vi "UHR-Fleezers Control (host) - Avogadro v3.vi"() -> ()   [LabVIEW 2014] (continued)
          n945 = disable-structure shown="Disabled" {
            disable-tunnel: [w1522 _] -> w1520
            disable-tunnel: w1519 -> [w1521 _]
            frame Disabled {
              n946 = call-poly <vilib>:"DB Tools Open Connection.vi"("connection information"=w1521) -> ("connection reference"=w1522:T28)  [unwired: 7 in, 1 out]
            }
            frame Enabled {
            }
          }
          "connection reference" <- w1520
          n947 = local write "connection reference"(w1520) -> ()
          n948 = local write "Database link"(w1519) -> ()
        }
        frame #3 {
          # "Load active calibration to fpga"
          n949 = local read "Base N trap periods"() -> (w1524:u32)
          n950 = local read "T1 Osc Enable"() -> (w1523:bool)
          n951 = property on="T1 Osc Enable" class="Bool (strict)"("Val(Sgnl)"=w1523) -> ()  [unwired: 2 in, 2 out]
          n952 = property on="Base N trap periods" class="DigNum (strict)"("Val(Sgnl)"=w1524) -> ()  [unwired: 2 in, 2 out]
        }
      }
    }
    frame #4 {
      # "Set FIFO size and run FPGA"
      n953 = local read "FPGA error out"() -> (w1526:errorcluster)
      n954 = xnode "Invoke Method"("FPGA VI Reference In"=w1527, "error in"=w1526, "Requested Depth"="Trap AI FIFO Depth") -> ("FPGA VI Reference Out"=w1531:T41, "error out"=w1532:errorcluster)  [unwired: 1 out]
      n955 = xnode "Invoke Method"("FPGA VI Reference In"=w1531, "error in"=w1532, "Requested Depth"="Trap Position FIFO Depth") -> ("FPGA VI Reference Out"=w1529:T41, "error out"=w1528:errorcluster)  [unwired: 1 out]
      n956 = xnode "Invoke Method"("FPGA VI Reference In"=w1529, "error in"=w1528) -> ("error out"=w1525:errorcluster)  [unwired: 1 in, 1 out]
      n957 = local write "FPGA error out"(w1525) -> ()
    }
    frame #5 {
      # "Adjust FPGA timing loop phases"
      n958 = flat-sequence "Initial FPGA Loop Relative Phase Adjustment" {
        tunnel: "Initial Phase Adjustment (AI1)" -> [w1568]
        tunnel: "Initial Phase Adjustment (Vortran)" -> [w1567]
        tunnel: "Initial Phase Adj. (MCL)" -> [w1566]
        tunnel: [w1569] -> w1552
        tunnel: [w1565] -> w1551
        tunnel: "Initial Phase Adjustment (APD Acq)" -> [w1564]
        tunnel: "Initial Phase Adjustment (APD 1 Gate)" -> [w1563]
        tunnel: "Initial Phase Adjustment (Green FB)" -> [w1562]
        tunnel: "Initial Phase Adjustment (GI) 2" -> [w1561]
        tunnel: "Initial Phase Adjustment (APD 2 Gate)" -> [w1560]
        tunnel: "Initial Phase Adjustment (RI)" -> [w1559]
        tunnel: "Initial Phase Adjustment (BI DO)" -> [w1558]
        tunnel: "Initial Phase Adjustment (BI AO)" -> [w1557]
        tunnel: "Initial Phase Adjustment (APD 3 Gate)" -> [w1556]
        tunnel: w1537 -> [w1555]
        tunnel: "Initial Phase Adjustment (EMCCD Gate)" -> [w1553]
        tunnel: w1552 -> [w1571]
        tunnel: [w1572] -> w1550
        tunnel: w1551 -> [w1572]
        tunnel: [w1571] -> w1549
        tunnel: w1550 -> [w1576]
        tunnel: w1549 -> [w1575]
        tunnel: [w1574] -> w1536
        frame #0 {
          n959 = local read "FPGA error out"() -> (w1554:errorcluster)
          n960 = xnode "Read/Write Control"("FPGA VI Reference In"=w1555, "error in"=w1554, "Phase count adjustment"=w1568, "Phase count adjustment (GI)"=w1567, "Phase count adjustment (MCL)"=w1566, "Phase Count Adjustment (APD Acq)"=w1564, "Phase count adjustment (APD 1 Gate)"=w1563, "Phase count adjustment (APD 2 Gate)"=w1560, "Phase count adjustment (Green FB)"=w1562, "Phase count adjustment (GI) 2"=w1561, "Phase count adjustment (RI)"=w1559, "Phase count adjustment (BI AO)"=w1557, "Phase count adjustment (BI D)"=w1558, "Phase count adjustment (APD 3 Gate)"=w1556, "Phase Count Adjustment EMCCD Gate"=w1553) -> ("FPGA VI Reference Out"=w1565:T41, "error out"=w1569:errorcluster)
        }
        frame #1 {
          n961 = Wait (ms)(milliseconds to wait=u32 100) -> ()  [unwired: 1 out]
        }
        frame #2 {
          w1573 = TRUE
          n962 = xnode "Read/Write Control"("FPGA VI Reference In"=w1576, "error in"=w1575, "+ phase"=w1573, "+ phase (GI)"=w1573, "+ phase (MCL)"=w1573, "+ phase (APD Acq)"=w1573, "+ phase (APD 1 Gate)"=w1573, "+ phase (APD 2 Gate)"=w1573, "+ phase (Green FB)"=w1573, "+ phase (GI) 2"=w1573, "+ phase (RI)"=w1573, "+ phase (BI AO)"=w1573, "+ phase (BI D)"=w1573, "+ phase (APD 3 Gate)"=w1573, "+ phase (EMCCD Gate)"=w1573) -> ("error out"=w1574:errorcluster)  [unwired: 1 out]
        }
      }
      n963 = local write "FPGA error out"(w1536) -> ()
    }
    frame #6 {
      w1592 = 6.0  # clock mult.
      w1591 = 49152000.0  # TCXO frequ.
      w1596 = 6.0  # clock mult.
      w1597 = 49152000.0  # TCXO frequ.
      # "Added by ronen - definition of \nlimit frequencies when using dynamic feedback"
      # "Initialize trap RF synth board and set initial frequencies and amplitudes"
      n964 = local read "FPGA error out"() -> (w1577:errorcluster)
      n965 = call "set RF board frequency - interlace.vi"("Board 2 Frequency Limits"=w1603, "Board 1 Frequency Limits"=w1584, "error in"=w1577, "FPGA VI Reference In"=w1578, "Board 2 Frequency 3 (MHz)"="BD 2 Frequency 3 (MHz)", "Board 1 Frequency 3 (MHz)"="BD 1 Frequency 3 (MHz)", "Board 2 Frequency 2 (MHz)"="BD 2 Frequency 2 (MHz)", "Board 2 Frequency 1 (MHz)"="BD 2 Frequency 1 (MHz)", "Board 1 Frequency 2 (MHz)"="BD 1 Frequency 2 (MHz)", "Board 1 Frequency 1  (MHz)"="BD 1 Frequency 1 (MHz)") -> ("error out"=w1608:errorcluster, "FPGA VI Reference Out"=w1583:T41)
      n966 = Unbundle By Name(w1584) -> ("Maximum"=w1594:dbl, "Minimum"=w1585:dbl)
      n967 = call "set RF board amplitude - interlace.vi"("Board 2 Amplitude Limits"=w1605, "Board 1 Amplitude Limits"=w1604, "error in"=w1608, "FPGA VI Reference In"=w1583, "Board 2 Amplitude 3 (%)"="BD 2 Amplitude 3 (%)", "Board 1 Amplitude 3 (%)"="BD 1 Amplitude 3 (%)", "Board 2 Amplitude 2 (%)"="BD 2 Amplitude 2 (%)", "Board 2 Amplitude 1 (%)"="BD 2 Amplitude 1 (%)", "Board 1 Amplitude 2 (%)"="BD 1 Amplitude 2 (%)", "Board 1 Amplitude 1 (%)"="BD 1 Amplitude 1 (%)") -> ("error out"=w1580:errorcluster)  [unwired: 1 out]
      n968 = Multiply(x=w1585, y=1000000.0) -> (x*y=w1589:dbl)
      n969 = Multiply(x=w1594, y=1000000.0) -> (x*y=w1599:dbl)
      n970 = Scale By Power Of 2(n=48, x=w1589) -> (x*2^n=w1587:dbl)
      n971 = Subtract(x="BD 1 Frequency 1 (MHz)", y="BD 1 Frequency 2 (MHz)") -> (x-y=w1615:dbl)
      n972 = Subtract(x="BD 2 Frequency 1 (MHz)", y="BD 2 Frequency 2 (MHz)") -> (x-y=w1616:dbl)
      n973 = Scale By Power Of 2(n=48, x=w1599) -> (x*2^n=w1601:dbl)
      n974 = Multiply(x=w1591, y=w1592) -> (x*y=w1593:dbl)
      n975 = Multiply(x=w1597, y=w1596) -> (x*y=w1595:dbl)
      n976 = Square(x=w1616) -> (x^2=w1618:dbl)
      n977 = Square(x=w1615) -> (x^2=w1617:dbl)
      n978 = Divide(x=w1587, y=w1593) -> (x/y=w1588:dbl)
      n979 = Divide(x=w1601, y=w1595) -> (x/y=w1600:dbl)
      n980 = Add(x=w1617, y=w1618) -> (x+y=w1619:dbl)
      n981 = To Unsigned Quad Integer(1:w1588) -> (0:w1581:u64)
      n982 = To Unsigned Quad Integer(1:w1600) -> (0:w1582:u64)
      n983 = Square Root(x=w1619) -> (sqrt(x)=w1620:dbl)
      n984 = local write "Trap Delta (MHz)"(w1620) -> ()
      n985 = xnode "Read/Write Control"("FPGA VI Reference In"=w1583, "error in"=w1580, "FB Max Frequency"=w1582, "FB Min frequency"=w1581) -> ("error out"=w1579:errorcluster)  [unwired: 1 out]
      n986 = local write "FPGA error out"(w1579) -> ()
    }
    frame #7 {
      n987 = flat-sequence {
        frame #0 {
          n988 = local read "Trap 1 (ON/OFF)"() -> (w1625:bool)
          n989 = local write "Saving..."(FALSE ("Saving Data")) -> ()
          n990 = local write "Stop All"(FALSE ("Stop All")) -> ()
          n991 = local write "Index"(1.0 ("Index")) -> ()
          n992 = property on="Trap 1 ON" class="Bool (strict)"("Value"=w1625) -> ()  [unwired: 2 in, 2 out]
          "Manipulating Trap" <- FALSE ("Manipulating Trap")
        }
        frame #1 {
          n993 = local read "Trap 2 (ON/OFF)"() -> (w1630:bool)
          n994 = Wait (ms)(milliseconds to wait=u32 10) -> ()  [unwired: 1 out]
          n995 = property on="Trap 2 ON" class="Bool (strict)"("Val(Sgnl)"=w1630) -> ()  [unwired: 2 in, 2 out]
        }
        frame #2 {
          n996 = local read "Scan Range (nm)"() -> (w1632:dbl)
          n997 = call "Update messages.vi"("Message to add"="UHR-Fleezers ready.", "Old message string"="") -> ("New message string"=w1635:string)
          n998 = local write "Messages"(w1635) -> ()
          n999 = property on="Scan Range (nm)" class="DigNum (strict)"("Val(Sgnl)"=w1632) -> ()  [unwired: 2 in, 2 out]
        }
      }
    }
    frame #8 {
      w1666 = 0
      w1665 = 2
      w1664 = 0
      w1661 = 3
      w1660 = 2
      w1659 = 5
      w1657 = 1
      w1656 = 2
      w1698 = u32 0
      w1704 = cluster{u32, u32} {16777238, 16777238}
      w1699 = 0.0
      # "Initialize the multi-MCL offset array"
      # "Initialize valves"
      # "Cursor control of trap\n3"
      # "Graph of positions and displacements in 2D"
      n1000 = local read "MCL offset scanning range (V)"() -> (w1685:T4)
      n1001 = control-ref of="Positions \nand displacements"() -> (w1636:refnum<vi>)
      n1002 = local read "Offset file step size"() -> (w1688:dbl)
      n1003 = Divide(x=30.0, y=w1688) -> (x/y=w1679:dbl)
      n1004 = call "start_stage_trackball.vi"("Enum"=T46."Trackball XY", "Stage Controller port"=w1692) -> ("error out"=w1690:errorcluster)  [unwired: 1 in, 1 out]
      n1005 = Initialize Array(0.0, w1679) -> (w1686:dbl[])
      n1006 = call "Make Trap3 position array.vi"("MCL offset scanning range (V)"=w1685) -> ("X Data points"=w1678:u64, "Y data points"=w1681:u64)  [unwired: 3 out]
      n1007 = property on="Stage Control Serial Error" class="Clust (strict)"("Val(Sgnl)"=w1690) -> ()  [unwired: 2 in, 2 out]
      n1008 = Bundle(w1686, w1686, w1686, w1686, w1686, w1686) -> (w1683:T51)  [unwired: 1 in]
      n1009 = Multiply(x=w1681, y=w1678) -> (x*y=w1684:u64)
      n1010 = for {
        N: w1684 -> [_]
        tunnel: [w1715] -> w1682 mode=indexing
        tunnel: w1683 -> [w1715]
      }
      n1011 = Build Array("T1", "T2", "T3", "disp1", "disp2", "disp3", "junc1", "junc2", "junc3", "Mean Junc") -> (w1677:string[])
      n1012 = property class="XYGraph (strict)"(reference=w1636, "Legend:Plots Shown"=10, "XScale.Maximum"=7900.0, "XScale.Minimum"=1000.0, "YScale.Maximum"=400.0, "YScale.Minimum"=-3200.0, "Frame Color"=u32 9868950) -> (reference out=w1644:refnum<vi>)  [unwired: 1 in, 1 out]
      n1013 = Reshape Array(w1682, w1678, w1681) -> (w1680:T52)
      n1014 = local write "Multi-MCL offset array"(w1680) -> ()
      n1015 = Build Array(u32 16711680, u32 16711680, u32 16711680, u32 40779, u32 40779, u32 40779, u32 16711898, u32 16711898, u32 16711898, u32 16860) -> (w1655:u32[])
      n1016 = Build Array(w1656, w1656, w1656, w1657, w1657, w1657, w1657, w1657, w1657, w1657) -> (w1658:i32[])
      n1017 = Build Array(w1659, w1659, w1659, w1660, w1660, w1660, w1661, w1661, w1661, 5) -> (w1663:i32[])
      n1018 = Build Array(w1664, w1664, w1664, w1665, w1665, w1665, w1666, w1666, w1666, w1666) -> (w1667:i32[])
      n1019 = for {
        tunnel: w1644 -> [w1714]
        tunnel: w1655 -> [w1712] mode=indexing
        tunnel: w1658 -> [w1711] mode=indexing
        tunnel: w1663 -> [w1710] mode=indexing
        tunnel: w1667 -> [w1709] mode=indexing
        tunnel: w1677 -> [w1707] mode=indexing
        i -> [w1713]
        n1020 = property class="XYGraph (strict)"(reference=w1714, "Active Plot"=w1713) -> (reference out=w1708:refnum<vi>)  [unwired: 1 in, 1 out]
        n1021 = property class="XYGraph (strict)"(reference=w1708, "Plot.Fill/Pt. Color"=w1712, "Plot.Point Style"=w1711, "Plot.Line Width"=w1710, "Plot.Plot Interpolation"=w1709, "Plot.Plot Name"=w1707) -> ()  [unwired: 1 in, 2 out]
      }
      n1022 = control-ref of="Piezo trap cursor control"() -> (w1700:refnum<vi>)
      n1023 = property class="XYGraph (strict)"(reference=w1700, "XScale.Maximum"=10.0, "XScale.Minimum"=w1699, "YScale.Maximum"=w1699, "YScale.Minimum"=-10.0, "Plot Area Colors"=w1704, "Frame Color"=u32 9868950, "XScale.GridColors"=w1704, "YScale.GridColors"=w1704, "Cursor.Cursor Color"=u32 16711680, "Active Cursor"=w1698, "Cursor.CursorMode"=w1698) -> ()  [unwired: 1 in, 2 out]
      n1024 = call "hamilton_controller.vi"("VISA resource name in"="Visa resource for valves", "action"=T49."CONNECT") -> ("error out"=w1697:errorcluster, "VISA resource name out"=w1694:refnum<visa-resource-name>)  [unwired: 8 in]
      n1025 = call "hamilton_controller.vi"("VISA resource name in"=w1694, "error in"=w1697, "action"=T49."INITIALIZE VALVES") -> ("error out"=w1706:errorcluster)  [unwired: 7 in, 1 out]
    }
    frame #9 {
      # "Wait 5 s for all the event loops still being executed to finish."
      n1026 = Wait (ms)(milliseconds to wait=u32 5000) -> ()  [unwired: 1 out]
      n1027 = local read "FPGA error out"() -> (w1717:errorcluster)
    }
  }
  n1028 = node-c288() -> (w31:T43)  [unwired: 4 out]
  n1029 = disable-structure shown="Disabled" {
    frame Disabled {
      n1030 = while "Duncan's play event loop" {
        stop <- w1721 stop-if-true
        n1031 = Create User Event(user event datatype=TRUE ("Boolean")) -> (user event=w1722:refnum<user-event>)  [unwired: 1 in, 1 out]
        n1032 = Create User Event(user event datatype=TRUE ("Boolean")) -> (user event=w1728:refnum<user-event>)  [unwired: 1 in, 1 out]
        n1033 = global write "Global for fluorescence simulation mean (30 samples), (power series).vi" "Red Signal"(w1722) -> ()
        n1034 = global write "Global for fluorescence simulation mean (30 samples), (power series).vi" "Green Signal"(w1728) -> ()
        n1035 = register-events(w1728, w1722) -> (reference out=w1727:refnum<event-registration>)  [unwired: 2 in, 1 out]
        n1036 = event shown="[1] \"Start assembly line\": Value Change" {
          selector: w1727 -> [_ _ _ _]
          dyn-events: _ -> [_ _ _ _]
          timeout: 100 -> [_ _ _ _]
          event Timeout {
            n1037 = event-data() -> ()  [unwired: 1 in, 2 out]
          }
          event "Start assembly line": Value Change {
            n1038 = event-data() -> ("OldVal"=w1730:bool)  [unwired: 1 in, 4 out]
            n1039 = case shown="True" w1730 {
              selector: w1730 -> [_ w1731]
              frame False {
              }
              frame True {
                n1040 = property on="Move to Position 3" class="Bool (strict)"("Val(Sgnl)"=w1731) -> ()  [unwired: 2 in, 2 out]
                n1041 = case shown="1" "Numeric" {
                  frame 0, Default {
                  }
                  frame 1 {
                    n1042 = property on="Vortran Laser ON" class="Bool (strict)"("Val(Sgnl)"=TRUE ("Value (Signaling)")) -> ()  [unwired: 2 in, 2 out]
                  }
                  frame 2 {
                    n1043 = property on="Red Laser ON" class="Bool (strict)"("Val(Sgnl)"=TRUE) -> ()  [unwired: 2 in, 2 out]
                  }
                }
              }
            }
          }
          event User Event {
            n1044 = event-data() -> ("Boolean"=w1735:bool)  [unwired: 1 in, 3 out]
            "Green Fluorophore" <- w1735
            n1045 = property on="Start assembly line" class="Bool"("Val(Sgnl)"=w1735) -> ()  [unwired: 2 in, 2 out]
          }
          event User Event {
            n1046 = event-data() -> ("Boolean"=w1736:bool)  [unwired: 1 in, 3 out]
            "Red Fluorophore" <- w1736
            n1047 = property on="Start assembly line" class="Bool"("Val(Sgnl)"=w1736) -> ()  [unwired: 2 in, 2 out]
          }
        }
        n1048 = property on="Get Fluorophore" class="Bool (strict)"("Val(Sgnl)"="Get Fluorophore") -> ()  [unwired: 2 in, 2 out]
        n1049 = Wait (ms)(milliseconds to wait=u32 100) -> ()  [unwired: 1 out]
        n1050 = local read "Stop All"() -> (w1720:bool)
        n1051 = Or(x=w1720, y="stop") -> (x .or. y?=w1721:bool)
      }
    }
    frame Enabled {
    }
  }
  n1052 = timed-loop "Rough control of MCL mirror stage (debugging)" {
    tunnel: [w1739] -> w71
    timing: w31 -> [_]
    timing-out: [_] -> w30
    tunnel: w26 -> [w1737]
    stop <- w1739 stop-if-true
    n1053 = node-c288() -> ()  [unwired: 2 out]
    n1054 = case shown="1" "MCL Mode" {
      tunnel: w1737 -> [_ w1742 w1789]
      frame 0, Default {
      }
      frame 1 {
        n1055 = node-c288() -> (w1744:T43)  [unwired: 4 out]
        n1056 = timed-loop "Oscillate MCL mirror" {
          timing: w1744 -> [_]
          timing-out: [_] -> w1743
          tunnel: w1742 -> [w1745]
          i -> [w1783]
          stop <- w1746 stop-if-true
          n1057 = node-c288() -> (w1782:i64)  [unwired: 1 out]
          n1058 = Multiply(x="AO1", y=32767.0) -> (x*y=w1778:dbl)
          n1059 = Multiply(x="AO2", y=32767.0) -> (x*y=w1773:dbl)
          n1060 = Divide(x=w1778, y=10.0) -> (x/y=w1779:dbl)
          n1061 = Divide(x=w1773, y=10.0) -> (x/y=w1774:dbl)
          n1062 = To Word Integer(number=w1779) -> (16bit integer=w1771:i16)
          n1063 = To Word Integer(number=w1774) -> (16bit integer=w1770:i16)
          n1064 = Divide(x=w1782, y=i64 1000) -> (x/y=w1753:dbl)
          n1065 = Multiply(x=w1753, y=w1783) -> (x*y=w1764:dbl)
          n1066 = Multiply(x="Osc. freq. (Hz) 2", y=6.283185307179586) -> (x*y=w1765:dbl)
          n1067 = Multiply(x=w1765, y=w1764) -> (x*y=w1763:dbl)
          n1068 = Sine(x=w1763) -> (sin(x)=w1762:dbl)
          n1069 = Multiply(x=w1762, y="Osc. amp. (V)") -> (x*y=w1760:dbl)
          n1070 = Add(x=w1760, y="Osc. center (V)") -> (x+y=w1758:dbl)
          n1071 = Divide(x=w1758, y=10.0) -> (x/y=w1756:dbl)
          n1072 = Multiply(x=w1756, y=32767.0) -> (x*y=w1751:dbl)
          n1073 = Select(t=w1751, s="Scan axis", f=w1771) -> (s? t:f=w1769:dbl)
          n1074 = Select(t=w1770, s="Scan axis", f=w1751) -> (s? t:f=w1768:dbl)
          n1075 = local read "MCL Mode"() -> (w1750:u16)
          n1076 = Not Equal?(x=w1750, y=u16 1) -> (x != y?=w1747:bool)
          n1077 = local read "Stop All"() -> (w1748:bool)
          n1078 = xnode "Read/Write Control"("FPGA VI Reference In"=w1745, "AO1 (Y)"=w1769, "AO2 (X)"=w1768) -> ()  [unwired: 1 in, 2 out]
          n1079 = Compound Arithmetic op=OR(w1748, w1747) -> (w1746:bool)
          n1080 = node-c288() -> ()  [unwired: 2 out]
        }
        n1081 = node-c288(w1743) -> ()  [unwired: 1 out]
      }
      frame 2 {
        n1082 = case shown="True" "Start Scan" {
          tunnel: w1789 -> [_ w1791]
          frame False {
          }
          frame True {
            n1083 = Subtract(x="End (V)", y="Begin (V)") -> (x-y=w1798:dbl)
            n1084 = Decrement(x="N Points") -> (x-1=w1797:dbl)
            n1085 = Divide(x=w1798, y=w1797) -> (x/y=w1795:dbl)
            n1086 = for {
              N: "N Points" -> [_]
              tunnel: "Begin (V)" -> [w1814]
              tunnel: [w1806] -> w1801 mode=indexing
              tunnel: w1795 -> [w1805]
              tunnel: [w1803] -> w1794 mode=indexing
              tunnel: w1791 -> [w1802]
              i -> [w1813]
              n1087 = Multiply(x=w1805, y=w1813) -> (x*y=w1812:dbl)
              n1088 = Add(x=w1814, y=w1812) -> (x+y=w1809:dbl)
              n1089 = local read "Scan axis"() -> (w1804:bool)
              n1090 = local read "AO1"() -> (w1811:dbl)
              n1091 = local read "AO2"() -> (w1810:dbl)
              n1092 = Select(t=w1809, s=w1804, f=w1811) -> (s? t:f=w1808:dbl)
              n1093 = Select(t=w1810, s=w1804, f=w1809) -> (s? t:f=w1807:dbl)
              n1094 = flat-sequence {
                tunnel: w1808 -> [w1818]
                tunnel: w1807 -> [w1817]
                tunnel: w1802 -> [w1815]
                tunnel: [w1828] -> w1806
                tunnel: [w1827] -> w1803
                frame #0 {
                  w1821 = 10.0 ("y")
                  w1816 = 32767.0 ("y")
                  n1095 = Multiply(x=w1818, y=w1816) -> (x*y=w1824:dbl)
                  n1096 = Multiply(x=w1817, y=w1816) -> (x*y=w1822:dbl)
                  n1097 = Divide(x=w1824, y=w1821) -> (x/y=w1825:dbl)
                  n1098 = Divide(x=w1822, y=w1821) -> (x/y=w1823:dbl)
                  n1099 = To Word Integer(number=w1825) -> (16bit integer=w1819:i16)
                  n1100 = To Word Integer(number=w1823) -> (16bit integer=w1820:i16)
                  n1101 = xnode "Read/Write Control"("FPGA VI Reference In"=w1815, "AO1 (Y)"=w1819, "AO2 (X)"=w1820) -> ()  [unwired: 1 in, 2 out]
                }
                frame #1 {
                  n1102 = Wait (ms)(milliseconds to wait="DAQ Delay (ms)") -> ()  [unwired: 1 out]
                }
                frame #2 {
                  n1103 = local read "Slow mean"() -> (w1828:dbl)
                  n1104 = local read "Sigma"() -> (w1827:dbl)
                }
              }
            }
            n1105 = Bundle("Begin (V)"="Begin (V)", w1795, w1801) -> (→"MCL Scan":cluster{"Begin (V)":dbl, dbl, dbl[]})  [unwired: 1 out]
            n1106 = Bundle("Begin (V)"="Begin (V)", w1795, w1794) -> (→"MCL Scan 2":cluster{"Begin (V)":dbl, dbl, dbl[]})  [unwired: 1 out]
          }
        }
      }
    }
    n1107 = local read "Stop All"() -> (w1739:bool)
    n1108 = node-c288() -> ()  [unwired: 2 out]
  }
  n1109 = node-c288(w30) -> ()  [unwired: 1 out]
  n1110 = node-c288(2 ("Processor")) -> (w62:T43)  [unwired: 3 out]
  n1111 = timed-loop "Basic control parameters (all FPGA settings, other basic controls)" {
    shift-right: [w1836] -> _
    shift-left: errorcluster {"status"=FALSE, "code"=0, "source"=""} ("error out") -> [_]
    tunnel: [w1835] -> _
    timing: w62 -> [_]
    timing-out: [_] -> w61
    tunnel: w44 -> [w1834]
    tunnel: w40 -> [w1833]
    tunnel: w39 -> [w1832]
    tunnel: w38 -> [w1831]
    tunnel: w37 -> [w1830]
    tunnel: w26 -> [w1829]
    stop <- w1835 stop-if-true
    n1112 = node-c288() -> ()  [unwired: 2 out]
    n1113 = event shown="[22] \"Laser choice 0\", \"Laser choice 1\", \"Laser choice 2\", \"FL interlace ON count 0\", \"Fl interlace ON count 1\", \"FL interlace ON count 2\", \"FL interlace OFF count 0\", \"FL interlace OFF count 1\", \"FL interlace OFF count 2\": Value Change" {
      selector: _ -> [_ _ _ _ _ _ _ _ _ _ _ _ _ _ _ _ _ _ _ _ _ _ _ _ _ _ _ _ _ _ _ _ _ _ _ _ _ _ _ _ _ _ _ _ _ _ _ _ _ _ _ _ _ _ _ _ _ _ _ _ _ _ _ _ _ _ _ _ _ _ _ _ _ _ _ _ _ _ _ _ _ _ _ _ _ _ _ _ _ _ _ _ _ _ _ _]
      dyn-events: _ -> [_ _ _ _ _ _ _ _ _ _ _ _ _ _ _ _ _ _ _ _ _ _ _ _ _ _ _ _ _ _ _ _ _ _ _ _ _ _ _ _ _ _ _ _ _ _ _ _ _ _ _ _ _ _ _ _ _ _ _ _ _ _ _ _ _ _ _ _ _ _ _ _ _ _ _ _ _ _ _ _ _ _ _ _ _ _ _ _ _ _ _ _ _ _ _ _]
      timeout: _ -> [_ _ _ _ _ _ _ _ _ _ _ _ _ _ _ _ _ _ _ _ _ _ _ _ _ _ _ _ _ _ _ _ _ _ _ _ _ _ _ _ _ _ _ _ _ _ _ _ _ _ _ _ _ _ _ _ _ _ _ _ _ _ _ _ _ _ _ _ _ _ _ _ _ _ _ _ _ _ _ _ _ _ _ _ _ _ _ _ _ _ _ _ _ _ _ _]
      tunnel: [w1876 _ _ _ w1903 _ _ _ _ _ _ _ w2009 _ _ w2100 w2102 w2109 w2111 w2181 _ w2223 _ w2260 w2288 w2313 w2340 w2366 w2395 _ w2400 w2494 w2498 w2535 _ w2628 w2631 w2634 w2644 w2647 _ w2654 _ _ _ _ _ _ _ _ _ _ _ _ _ _ _ _ _ _ _ w3199 _ _ _ _ w3236 _ _ _ _ _ _ _ _ _ _ _ _ _ _ _ _ _ _ _ _ _ _ _ _ _ _ _ _ _] -> w1836
      tunnel: [_ _ _ _ _ _ _ _ _ _ w1988 _ _ _ _ _ _ _ _ _ _ _ _ _ _ _ _ _ _ _ _ _ _ _ _ _ _ _ _ _ _ _ _ _ _ _ _ _ _ _ _ _ _ _ _ _ _ _ _ _ _ _ _ _ _ _ _ _ _ _ _ _ _ _ _ _ _ _ _ _ _ _ _ _ _ _ _ _ _ _ _ _ _ _ _ _] -> w1835
      tunnel: [_ _ _ _ _ _ _ _ "Round T1 X" _ _ _ _ _ _ _ _ _ _ _ _ _ _ _ _ _ _ _ _ _ _ _ _ _ _ _ _ _ _ _ _ _ _ _ _ _ _ _ _ _ _ _ _ _ _ _ _ _ _ _ _ _ _ _ _ _ _ _ _ _ _ _ _ _ _ _ _ _ _ _ _ _ _ _ _ _ _ _ _ _ _ _ _ _ _ _] -> _
      tunnel: [_ _ _ "Adjust Scale\nto Mean" _ _ _ _ _ _ _ _ _ _ _ _ _ _ _ _ _ _ _ _ _ _ _ _ _ _ "Test ttrig" _ _ _ _ _ _ _ _ _ _ _ _ _ _ _ _ _ _ _ _ w2946 w3010 w3057 w3106 _ _ _ _ _ _ _ _ _ _ _ _ _ _ _ _ _ _ _ _ _ _ _ _ _ _ _ _ _ _ _ _ _ _ _ _ _ _ _ _ _] -> _
      tunnel: [_ _ _ _ _ _ _ _ _ "Round T2 X" _ "Delayed Interlace Start" _ _ _ _ _ _ _ _ _ _ _ _ _ _ _ _ _ _ _ _ _ _ _ _ _ _ _ _ _ _ _ _ _ _ _ _ _ _ _ _ _ _ _ _ _ _ _ _ _ _ _ _ _ _ _ _ _ _ _ _ _ _ _ _ _ _ _ _ _ _ _ _ _ _ _ _ _ _ _ _ _ _ _ _] -> _
      tunnel: w1834 -> [_ _ _ _ _ _ _ _ _ _ _ _ _ _ _ _ _ _ _ _ _ _ _ _ _ _ _ _ _ _ _ _ _ _ _ _ _ _ _ _ _ _ _ _ _ _ _ w2916 w2924 w2931 w2937 w2945 _ _ w3105 _ _ _ _ _ _ _ _ _ _ _ _ _ _ _ _ _ _ _ _ _ _ _ _ _ _ _ _ _ _ _ _ _ _ _ _ _ _ _ _ _]
      tunnel: w1833 -> [_ _ _ _ _ _ _ _ _ _ _ _ _ _ _ _ _ _ _ _ _ _ _ _ _ _ _ _ _ _ _ _ _ _ _ _ _ _ _ _ _ _ _ _ _ w2803 _ _ _ _ _ _ w3009 _ _ w3112 _ w3124 _ w3140 _ _ _ _ _ _ _ _ _ _ _ _ _ _ _ _ _ _ _ _ _ _ _ _ _ _ _ _ _ _ _ _ _ _ _ _]
      tunnel: w1832 -> [_ _ _ _ _ _ _ _ _ _ _ _ _ _ _ _ _ _ _ _ _ _ _ _ _ _ _ _ _ _ _ _ _ _ _ _ _ _ _ _ _ _ _ _ _ _ _ _ _ _ _ _ _ _ _ _ _ _ _ _ _ _ _ _ _ _ _ _ _ _ _ _ _ _ _ _ _ _ _ _ _ _ _ _ _ _ _ _ _ _ _ _ _ _ _ _]
      tunnel: w1831 -> [_ _ _ _ _ _ _ _ _ _ _ _ _ _ _ _ _ _ _ _ _ _ _ _ _ _ _ _ _ _ _ _ _ _ _ _ _ _ _ _ _ _ w2665 _ _ _ _ _ _ _ _ _ _ w3056 _ _ w3118 _ w3132 _ w3166 _ _ _ _ _ _ _ _ _ _ _ _ _ _ _ _ _ _ _ _ _ _ _ _ _ _ _ _ _ _ _ _ _ _ _]
      tunnel: w1830 -> [_ _ _ _ _ _ _ _ _ _ _ _ _ _ _ _ _ _ _ _ _ _ _ _ _ _ _ _ _ _ _ _ _ _ _ _ _ _ _ _ _ _ _ _ _ _ _ _ _ _ _ _ _ _ _ _ _ _ _ _ _ _ _ _ _ _ _ _ _ _ _ _ _ _ _ _ _ _ _ _ _ _ _ _ _ _ _ _ _ _ _ _ _ _ _ _]
      tunnel: w1829 -> [w1839 _ _ _ w1902 _ w1928 _ _ _ _ _ w2000 _ _ w2084 w2101 w2108 w2110 w2146 _ w2212 w2247 w2258 w2270 w2295 w2323 w2343 w2371 w2396 w2398 w2402 w2495 w2499 _ w2625 w2629 w2632 w2642 w2645 _ w2653 _ _ w2748 _ _ _ _ _ _ _ _ _ _ _ _ _ _ _ _ w3192 _ w3213 _ w3220 w3235 _ w3242 w3269 w3276 w3292 w3300 _ w3311 _ w3355 _ _ w3409 w3440 w3444 w3452 _ w3516 w3526 w3545 _ _ _ _ _ _ w3698 w3703 w3710]
      tunnel: [_ _ _ _ _ _ _ _ _ _ w1987 _ _ _ _ _ _ _ _ _ _ _ _ _ _ _ _ _ _ _ _ _ _ _ _ _ _ _ _ _ _ _ _ w2745 w2750 _ _ _ _ _ _ _ _ _ _ _ _ _ _ _ _ _ _ _ _ _ _ _ _ _ _ _ _ _ _ _ _ _ _ _ _ _ _ _ _ _ _ _ _ _ _ _ _ _ _ _] -> _
      event "AI Count (ticks)", "Sets to FIFO (Traps)", "Save ave N", "FPGA Ave.", "# Samples/channel", "N sets to save": Value Change {
        # "RG 18-01-16 Increased amount of elements to read for trap position, to add x and y for piezo trap"
        # "So that if 'Save ave N' is updated, the AOD scanning code updates too."
        n1114 = event-data() -> ()  [unwired: 6 out]
        n1115 = local read "AI Count (ticks)"() -> (w1860:u16)
        n1116 = Divide(x=40000000.0, y=w1860) -> (x/y=w1852:dbl)
        "AI rate (Hz)" <- w1852
        "Ave. Rate (Hz)" <- w1852
        n1117 = Reciprocal(x=w1852) -> (1/x=→"Ave. Period (s)":dbl)
        n1118 = Unbundle By Name("Sets to FIFO (Traps)") -> ("Set 1"=w1843:bool, "Set 2"=w1842:bool, "Set 3"=w1841:bool)
        n1119 = Divide(x=w1852, y="N Acq Sets (Traps + Fl.)") -> (x/y=w1873:dbl)
        "Data Rate (Hz)" <- w1873
        n1120 = Reciprocal(x=w1873) -> (1/x=→"Data Period (s)":dbl)
        n1121 = Boolean To (0,1)(Boolean="Sets to FIFO (Traps)") -> (0, 1=w1868:cluster{"Set 1":i16, "Set 2":i16, "Set 3":i16})
        n1122 = xnode "Read/Write Control"("FPGA VI Reference In"=w1839, "ai count"=w1860, "Set 1"=w1843, "Set 2"=w1842, "Set 3"=w1841, "N of AI1 Int Acq Sets"="N Acq Sets (Traps + Fl.)") -> ("error out"=w1876:errorcluster)  [unwired: 1 in, 1 out]
        n1123 = Cluster To Array(cluster=w1868) -> (array=w1867:i16[])
        n1124 = local read "Save ave N"() -> (w1872:dbl)
        n1125 = To Unsigned Long Integer(number=w1867) -> (unsigned 32bit integer=w1849:u32[])
        n1126 = Multiply(x=w1860, y="N Acq Sets (Traps + Fl.)") -> (x*y=w1858:u16)
        n1127 = local read "Scan steps (AOD)"() -> (w1869:u64)
        n1128 = Add Array Elements(numeric array=w1849) -> (sum=w1861:u32)
        "Trap Sets" <- w1861
        n1129 = Divide(x=w1873, y=w1872) -> (x/y=w1871:dbl)
        "Save Data Rate (Hz)" <- w1871
        n1130 = Reciprocal(x=w1871) -> (1/x=→"Save Data Period (s)":dbl)
        n1131 = property on="Scan steps (AOD)" class="DigNum (strict)"("Val(Sgnl)"=w1869) -> ()  [unwired: 2 in, 2 out]
        n1132 = Multiply(x=w1858, y="# Samples/trap") -> (x*y=w1856:u32)
        "Counts/DMA" <- w1856
        n1133 = property on="Trap Disp. Downsample" class="DigNum (strict)"("Maximum"="# Samples/trap") -> ()  [unwired: 2 in, 2 out]
        n1134 = Multiply(x=w1861, y="# Samples/trap") -> (x*y=w1850:u32)
        "# Samples/channel" <- w1850
        n1135 = Multiply(x=w1850, y=u32 8) -> (x*y=→"Trap AI Elements/DMA read":u32)
        n1136 = local read "APD Int. Count"() -> (w1857:u32)
        n1137 = Multiply(x=w1850, y=u32 5) -> (x*y=→"Trap Pos Elements/DMA read":u32)
        n1138 = Divide(x=w1856, y=w1857) -> (x/y=w1847:dbl)
        "APD Samples/FIFO Acq." <- w1847
        n1139 = Divide(x=w1856, y=40000000.0) -> (x/y=w1854:dbl)
        "DMA Update Period (s)" <- w1854
        n1140 = local read "Number of APDs"() -> (w1840:u8)
        n1141 = Multiply(x=w1840, y=w1847) -> (x*y=→"APD Elements/DMA read":dbl)
        n1142 = property on="APD Disp. Downsample" class="DigNum (strict)"("Maximum"=w1847) -> ()  [unwired: 2 in, 2 out]
        n1143 = local read "N sets to save"() -> (w1866:u32)
        n1144 = Multiply(x=w1854, y=w1866) -> (x*y=→"Total Time (s) 2":dbl)
        "FPGA Averaging" <- FALSE ("FPGA Averaging")
      }
      event "Remove Offset": Value Change {
        n1145 = event-data() -> ()  [unwired: 7 out]
        n1146 = local write "Remove Offset"(FALSE ("Remove Offset")) -> ()
        n1147 = local read "Bead Mean (nm)"() -> (w1878:dbl)
        n1148 = local read "Offset (nm)"() -> (w1879:dbl)
        n1149 = Add(x=w1878, y=w1879) -> (x+y=w1877:dbl)
        n1150 = local write "Offset (nm)"(w1877) -> ()
      }
      event "Detector Type": Value Change {
        n1151 = event-data() -> ()  [unwired: 7 out]
        n1152 = local read "AI labels"() -> (w1883:string[])
        n1153 = property on="High Res. Display" class="Ring (strict)"("Strings []"=w1883) -> ()  [unwired: 2 in, 2 out]
        n1154 = Build Array (concatenate)(w1883, "none") -> (w1884:string[])
        n1155 = property on="FFT 1 Choice 1" class="Ring (strict)"("Strings []"=w1884) -> ()  [unwired: 2 in, 2 out]
        n1156 = property on="FFT 1 Choice 2" class="Ring (strict)"("Strings []"=w1884) -> ()  [unwired: 2 in, 2 out]
        n1157 = property on="FFT 2 Choice 1" class="Ring (strict)"("Strings []"=w1884) -> ()  [unwired: 2 in, 2 out]
        n1158 = property on="FFT 2 Choice 2" class="Ring (strict)"("Strings []"=w1884) -> ()  [unwired: 2 in, 2 out]
        n1159 = Bundle("APD 1", "APD 2", "APD 3") -> (w1887:cluster{string, string, string})  [unwired: 1 out]
        n1160 = Cluster To Array(cluster=w1887) -> (array=w1885:string[])
        n1161 = Build Array (concatenate)(w1885, w1884) -> (w1889:string[])
        n1162 = Array Size(array=w1889) -> (size(s)=w1881:i32)
        n1163 = property on="Signals to Plot" class="LstBox (strict)"("Item Names"=w1889) -> ()  [unwired: 2 in, 2 out]
        n1164 = property on="Signals to Plot" class="LstBox (strict)"("Number of Rows"=w1881) -> ()  [unwired: 2 in, 2 out]
        n1165 = property on="All Signals" class="WFChart (strict)"("LegNumRows"=w1881) -> ()  [unwired: 2 in, 2 out]
      }
      event "Adjust Scale\nto Mean": Value Change {
        n1166 = event-data() -> ()  [unwired: 7 out]
        n1167 = local read "APD rates cluster"() -> (w1892:T2)
        n1168 = Unbundle By Name(w1892) -> ("APD 1 Rate (Hz)"=w1891:dbl)
        n1169 = Multiply(x=1000.0, y="Above (kHz)") -> (x*y=w1898:dbl)
        n1170 = Multiply(x=1000.0, y="Below (kHz)") -> (x*y=w1896:dbl)
        n1171 = Add(x=w1898, y=w1891) -> (x+y=w1893:dbl)
        n1172 = Subtract(x=w1891, y=w1896) -> (x-y=w1894:dbl)
        n1173 = property on="APD Chart" class="WFChart (strict)"("YScale.Minimum"=w1894) -> ()  [unwired: 2 in, 2 out]
        n1174 = property on="APD Chart" class="WFChart (strict)"("YScale.Maximum"=w1893) -> ()  [unwired: 2 in, 2 out]
      }
      event "Phase adj. (AI1)", "+ phase (AI1)", "- phase (AI1)": Value Change {
        n1175 = event-data() -> ()  [unwired: 7 out]
        n1176 = Negate(x="Phase adj. (AI1)") -> (-x=w1910:i16)
        n1177 = Select(t=w1910, s="- phase (AI1)", f="Phase adj. (AI1)") -> (s? t:f=w1909:i16)
        n1178 = xnode "Read/Write Control"("FPGA VI Reference In"=w1902, "Phase count adjustment"=w1909) -> ("FPGA VI Reference Out"=w1908:T41, "error out"=w1907:errorcluster)  [unwired: 2 in]
        n1179 = Or(x="- phase (AI1)", y="+ phase (AI1)") -> (x .or. y?=w1904:bool)
        n1180 = xnode "Read/Write Control"("FPGA VI Reference In"=w1908, "error in"=w1907, "+ phase"=w1904) -> ("error out"=w1903:errorcluster)  [unwired: 1 in, 1 out]
      }
      event "Signals to Plot": Double Click {
        w1922 = u32 9868950 ("Color Box")
        n1181 = event-data() -> ("Row"=w1913:i32)  [unwired: 9 out]
        n1182 = property on="All Signals" class="WFChart (strict)"("Active Plot"=w1913) -> (error out=w1912:errorcluster)  [unwired: 2 in, 1 out]
        n1183 = property on="All Signals" class="WFChart (strict)" props=["Plot", "Plot Color", "Plot", "Visible?"](error in=w1912) -> (error out=w1915:errorcluster, "Plot.Visible?"=w1914:bool)  [unwired: 1 in, 2 out]
        n1184 = Select(t=FALSE ("Plot.Visible"), s=w1914, f=TRUE ("Plot.Visible")) -> (s? t:f=w1917:bool)
        n1185 = property on="All Signals" class="WFChart (strict)"(error in=w1915, "Plot.Visible?"=w1917) -> (error out=w1916:errorcluster)  [unwired: 1 in, 1 out]
        n1186 = property on="All Signals" class="WFChart (strict)"(error in=w1916) -> (error out=w1918:errorcluster, "Plot.Plot Color"=w1919:u32)  [unwired: 1 in, 1 out]
        n1187 = property on="Signals to Plot" class="LstBox (strict)"(error in=w1918, "Active Row"=w1913) -> (error out=w1923:errorcluster)  [unwired: 1 in, 1 out]
        n1188 = Select(t=w1919, s=w1917, f=u32 0) -> (s? t:f=w1924:u32)
        n1189 = property on="Signals to Plot" class="LstBox (strict)"(error in=w1923, "CellFontColor"=w1924, "SelColor"=w1922, "CellBG"=w1922, "CellFontSize"=u32 20 ("Active Row:Cell Font:Size"), "CellFontBold"=TRUE ("Active Row:Cell Font:Bold")) -> ()  [unwired: 1 in, 2 out]
      }
      event "BD 1 Frequency 1 (MHz)", "BD 1 Frequency 2 (MHz)", "BD 1 Frequency 3 (MHz)", "BD 2 Frequency 1 (MHz)", "BD 2 Frequency 2 (MHz)", "BD 2 Frequency 3 (MHz)", "Trap Delta (MHz)", "Update all trap values": Value Change {
        # "This is so you can set trap frequencies\nvia local variables and then update\nall at once"
        n1190 = event-data() -> ("CtlRef"=w1932:refnum<vi>)  [unwired: 6 out]
        n1191 = control-ref of="Trap Delta (MHz)"() -> (w1931:refnum<vi>)
        n1192 = Equal?(x=w1931, y=w1932) -> (x = y?=w1930:bool)
        n1193 = local write "Update all trap values"(FALSE ("Update all trap values")) -> ()
        n1194 = case shown="False" "Oscillate Set 1" {
          tunnel: w1930 -> [w1946 _]
          tunnel: w1928 -> [w1944 _]
          frame False {
            n1195 = local read "BD 1 Frequency 2 (MHz)"() -> (w1942:dbl)
            n1196 = case shown="True" "Symmetric \nmanual\n motion" {
              tunnel: "Trap Delta (MHz)" -> [w1968 w1975]
              tunnel: [w1969 w1973] -> w1934
              tunnel: [w1967 w1971] -> w1936
              tunnel: w1942 -> [w1969 _]
              frame False {
                n1197 = Subtract(x=w1969, y=w1968) -> (x-y=w1967:dbl)
              }
              frame True {
                n1198 = Divide(x=w1975, y=2.0) -> (x/y=w1972:dbl)
                n1199 = Add(x=w1972, y="center Hz for  manual\nsymmetric motion") -> (x+y=w1973:dbl)
                n1200 = Subtract(x="center Hz for  manual\nsymmetric motion", y=w1972) -> (x-y=w1971:dbl)
              }
            }
            n1201 = local read "BD 1 Frequency 1 (MHz)"() -> (w1937:dbl)
            n1202 = Not(x="Symmetric \nmanual\n motion") -> (.not. x?=w1940:bool)
            n1203 = And(x=w1940, y="move Con X?") -> (x .and. y?=w1938:bool)
            n1204 = Subtract(x=w1937, y=w1936) -> (x-y=w1935:dbl)
            n1205 = Select(t=w1936, s=w1946, f=w1937) -> (s? t:f=w1945:dbl)
            n1206 = local read "Y RF Frequency Limits (MHz)"() -> (w1947:T27)
            n1207 = case shown="True" w1938 {
              tunnel: w1935 -> [_ w1966]
              frame False {
              }
              frame True {
                n1208 = property on="AOM X Cal (nm/MHz)" class="DigNum (strict)"() -> ("Value"=w1965:dbl)  [unwired: 2 in, 2 out]
                n1209 = property on="MCL Step Position Ratio" class="DigNum (strict)"() -> ("Value"=w1959:dbl)  [unwired: 2 in, 2 out]
                n1210 = Compound Arithmetic op=MULTIPLY(w1966, w1965, w1959) -> (w1964:dbl)
                n1211 = property on="MCL X Cal (nm/V)" class="DigNum (strict)"() -> ("Value"=w1963:dbl)  [unwired: 2 in, 2 out]
                n1212 = Divide(x=w1964, y=w1963) -> (x/y=w1962:dbl)
                n1213 = property on="AO2" class="Slide (strict)"() -> ("Value"=w1961:dbl)  [unwired: 2 in, 2 out]
                n1214 = Add(x=w1962, y=w1961) -> (x+y=w1960:dbl)
                n1215 = property on="AO2" class="Slide (strict)"("Val(Sgnl)"=w1960) -> ()  [unwired: 2 in, 2 out]
              }
            }
            n1216 = local read "X RF Frequency Limits (MHz)"() -> (w1948:T27)
            n1217 = local write "BD 1 Frequency 1 (MHz)"(w1945) -> ()
            n1218 = local read "BD 1 Frequency 3 (MHz)"() -> (w1957:dbl)
            n1219 = local read "BD 2 Frequency 1 (MHz)"() -> (w1951:dbl)
            n1220 = local read "BD 2 Frequency 2 (MHz)"() -> (w1950:dbl)
            n1221 = local read "BD 2 Frequency 3 (MHz)"() -> (w1958:dbl)
            n1222 = call "set RF board frequency - interlace.vi"("Board 2 Frequency Limits"=w1947, "Board 1 Frequency Limits"=w1948, "FPGA VI Reference In"=w1944, "Board 2 Frequency 3 (MHz)"=w1958, "Board 1 Frequency 3 (MHz)"=w1957, "Board 2 Frequency 2 (MHz)"=w1950, "Board 2 Frequency 1 (MHz)"=w1951, "Board 1 Frequency 2 (MHz)"=w1934, "Board 1 Frequency 1  (MHz)"=w1945) -> ()  [unwired: 1 in, 2 out]
            n1223 = Subtract(x=w1951, y=w1950) -> (x-y=w1955:dbl)
            n1224 = local write "BD 1 Frequency 2 (MHz)"(w1934) -> ()
            n1225 = Subtract(x=w1945, y=w1934) -> (x-y=w1956:dbl)
            n1226 = Square(x=w1955) -> (x^2=w1953:dbl)
            n1227 = Square(x=w1956) -> (x^2=w1954:dbl)
            n1228 = Add(x=w1954, y=w1953) -> (x+y=w1952:dbl)
            n1229 = Square Root(x=w1952) -> (sqrt(x)=w1949:dbl)
            n1230 = property on="Initial delta (MHz)" class="DigNum (strict)"("Val(Sgnl)"=w1949) -> ()  [unwired: 2 in, 2 out]
            n1231 = local write "Trap Delta (MHz)"(w1949) -> ()
          }
          frame True {
          }
        }
      }
      event "manual raster set": Value Change {
        n1232 = event-data() -> ()  [unwired: 7 out]
        n1233 = flat-sequence {
          frame #0 {
            n1234 = Replace Array Subset(array=u32[] [0] ("Index Values"), new element="manual raster set", index=0) -> (w1976:u32[])
            n1235 = property on="Saved AOD Raster Scan Parameter Sets" class="Arr (strict)"("Index Values"=w1976) -> ()  [unwired: 2 in, 2 out]
          }
          frame #1 {
            n1236 = property on="Load parameters" class="Bool (strict)"("Val(Sgnl)"=TRUE ("Value (Signaling)")) -> ()  [unwired: 2 in, 2 out]
          }
        }
      }
      event "Round T1 X": Value Change {
        n1237 = event-data() -> ()  [unwired: 7 out]
        n1238 = local read "BD 1 Frequency 1 (MHz)"() -> (w1983:dbl)
        n1239 = Round To Nearest(number=w1983) -> (nearest integer value=w1982:dbl)
        n1240 = property on="BD 1 Frequency 1 (MHz)" class="DigNum (strict)"("Val(Sgnl)"=w1982) -> ()  [unwired: 2 in, 2 out]
      }
      event "Round T2 X": Value Change {
        n1241 = event-data() -> ()  [unwired: 7 out]
        n1242 = local read "BD 1 Frequency 2 (MHz)"() -> (w1985:dbl)
        n1243 = Round To Nearest(number=w1985) -> (nearest integer value=w1984:dbl)
        n1244 = property on="BD 1 Frequency 2 (MHz)" class="DigNum (strict)"("Val(Sgnl)"=w1984) -> ()  [unwired: 2 in, 2 out]
      }
      event "Stop All": Value Change {
        n1245 = event-data() -> ()  [unwired: 7 out]
        n1246 = flat-sequence {
          tunnel: [w1991] -> w1989
          tunnel: [w1994] -> w1987
          tunnel: w1989 -> [w1994]
          tunnel: [TRUE] -> w1988
          frame #0 {
            n1247 = local read "Visa resource for valves"() -> (w1990:refnum<visa-resource-name>)
            n1248 = call "hamilton_controller.vi"("VISA resource name in"=w1990, "action"=T49."DISCONNECT") -> ("error out"=w1991:errorcluster)  [unwired: 8 in, 1 out]
          }
          frame #1 {
          }
        }
      }
      event "Delayed Interlace Start": Value Change {
        n1249 = event-data() -> ()  [unwired: 7 out]
        n1250 = flat-sequence {
          frame #0 {
            n1251 = Multiply(x="Delay to Interlace (s)", y=1000.0) -> (x*y=w1996:dbl)
            n1252 = Wait (ms)(milliseconds to wait=w1996) -> ()  [unwired: 1 out]
          }
          frame #1 {
            n1253 = property on="Laser interlacing mode" class="RadioBtnsControl (strict)"("Val(Sgnl)"=enum32{"Laser ON", "Laser OFF", "Interlace"}."Interlace" ("Value (Signaling)")) -> ()  [unwired: 2 in, 2 out]
          }
        }
      }
      event "BD 1 Amplitude 1 (%)", "BD 1 Amplitude 2 (%)", "BD 1 Amplitude 3 (%)", "BD 2 Amplitude 1 (%)", "BD 2 Amplitude 2 (%)", "BD 2 Amplitude 3 (%)", "Trap 1 ON", "Trap 2 ON", "Trap 3 ON", "Feedback On/Off", "All FB On/Off": Value Change {
        w2021 = i16 1 ("f")
        n1254 = event-data() -> ()  [unwired: 7 out]
        n1255 = local write "Trap 1 (ON/OFF)"("Trap 1 ON") -> ()
        n1256 = local write "Trap 2 (ON/OFF)"("Trap 2 ON") -> ()
        n1257 = Boolean To (0,1)(Boolean="Trap 3 ON") -> (0, 1=w2022:i16)
        n1258 = Boolean To (0,1)(Boolean="Trap 1 ON") -> (0, 1=w2023:i16)
        n1259 = Boolean To (0,1)(Boolean="Trap 2 ON") -> (0, 1=w2024:i16)
        n1260 = Select(t=w2024, s="Trap ON/OFF X or Y Amp?", f=w2021) -> (s? t:f=w2019:i16)
        n1261 = Select(t=w2023, s="Trap ON/OFF X or Y Amp?", f=w2021) -> (s? t:f=w2020:i16)
        n1262 = Select(t=w2022, s="Trap ON/OFF X or Y Amp?", f=w2021) -> (s? t:f=w2018:i16)
        n1263 = Select(t=w2021, s="Trap ON/OFF X or Y Amp?", f=w2024) -> (s? t:f=w2016:i16)
        n1264 = Select(t=w2021, s="Trap ON/OFF X or Y Amp?", f=w2023) -> (s? t:f=w2017:i16)
        n1265 = Select(t=w2021, s="Trap ON/OFF X or Y Amp?", f=w2022) -> (s? t:f=w2015:i16)
        n1266 = And(x="All FB On/Off", y="Feedback On/Off") -> (x .and. y?=w2013:cluster{"Set 1":bool, "Set 2":bool})
        n1267 = local read "BD 1 Amplitude 1 (%)"() -> (w2031:dbl)
        n1268 = local read "BD 1 Amplitude 2 (%)"() -> (w2030:dbl)
        n1269 = local read "BD 1 Amplitude 3 (%)"() -> (w2029:dbl)
        n1270 = Unbundle By Name(w2013) -> ("Set 1"=w2008:bool, "Set 2"=w2005:bool)
        n1271 = local read "Y RF Amplitude Limits (%)"() -> (w2001:T27)
        n1272 = local read "X RF Amplitude Limits (%)"() -> (w2002:T27)
        n1273 = local read "BD 2 Amplitude 1 (%)"() -> (w2032:dbl)
        n1274 = local read "BD 2 Amplitude 2 (%)"() -> (w2033:dbl)
        n1275 = local read "BD 2 Amplitude 3 (%)"() -> (w2034:dbl)
        n1276 = And(x="Trap 2 ON", y=w2005) -> (x .and. y?=w2003:bool)
        n1277 = And(x="Trap 1 ON", y=w2008) -> (x .and. y?=w2006:bool)
        n1278 = Multiply(x=w2020, y=w2031) -> (x*y=w2028:dbl)
        n1279 = Multiply(x=w2030, y=w2019) -> (x*y=w2026:dbl)
        n1280 = Multiply(x=w2029, y=w2018) -> (x*y=w2027:dbl)
        n1281 = Multiply(x=w2032, y=w2017) -> (x*y=w2035:dbl)
        n1282 = Multiply(x=w2033, y=w2016) -> (x*y=w2036:dbl)
        n1283 = Multiply(x=w2034, y=w2015) -> (x*y=w2037:dbl)
        n1284 = call "set RF board amplitude - interlace.vi"("Board 2 Amplitude Limits"=w2001, "Board 1 Amplitude Limits"=w2002, "FPGA VI Reference In"=w2000, "Board 2 Amplitude 3 (%)"=w2037, "Board 1 Amplitude 3 (%)"=w2027, "Board 2 Amplitude 2 (%)"=w2036, "Board 2 Amplitude 1 (%)"=w2035, "Board 1 Amplitude 2 (%)"=w2026, "Board 1 Amplitude 1 (%)"=w2028) -> ("error out"=w2010:errorcluster, "FPGA VI Reference Out"=w2011:T41)  [unwired: 1 in]
        n1285 = xnode "Read/Write Control"("FPGA VI Reference In"=w2011, "error in"=w2010, "FB On/Off Set 1"=w2006, "FB On/Off Set 2"=w2003) -> ("error out"=w2009:errorcluster)  [unwired: 1 out]
      }
      event "Load parameters": Value Change {
        n1286 = event-data() -> ()  [unwired: 7 out]
        n1287 = property on="Saved AOD Raster Scan Parameter Sets" class="Arr (strict)"() -> ("Index Values"=w2048:u32[])  [unwired: 2 in, 2 out]
        n1288 = Index Array(array=w2048, index=0) -> (element=w2045:u32)
        n1289 = local write "Load parameters"(FALSE ("Load parameters")) -> ()
        n1290 = Index Array(array="Saved AOD Raster Scan Parameter Sets", index=w2045) -> (element=w2044:T55)
        n1291 = Unbundle By Name(w2044) -> ("Scan Range AOD (nm) 2"=w2043:dbl, "Step Size AOD (nm) 2"=w2042:dbl, "Scan Speed AOD (nm/s) 2"=w2041:dbl, "Number of scans (AOD) 2"=w2040:u16)
        n1292 = flat-sequence {
          tunnel: w2043 -> [w2051]
          tunnel: w2042 -> [w2050]
          tunnel: w2041 -> [w2049]
          tunnel: w2040 -> [w2052]
          frame #0 {
            n1293 = local write "Scan Speed (nm/s)"(w2049) -> ()
            n1294 = local write "Scan Range (nm)"(w2051) -> ()
            n1295 = local write "Step Size (nm)"(w2050) -> ()
          }
          frame #1 {
            n1296 = property on="Number of F/B Scans (AOD)" class="DigNum (strict)"("Val(Sgnl)"=w2052) -> ()  [unwired: 2 in, 2 out]
          }
        }
      }
      event "Trap 1 (ON/OFF)", "Trap 2 (ON/OFF)": Value Change {
        n1297 = event-data() -> ()  [unwired: 7 out]
        n1298 = flat-sequence {
          tunnel: [w2062] -> w2057
          tunnel: w2057 -> [w2077]
          tunnel: [w2063] -> w2053
          frame #0 {
            n1299 = local read "Trap 1 ON"() -> (w2062:bool)
          }
          frame #1 {
            n1300 = Exclusive Or(1:w2077, 2:"Trap 1 (ON/OFF)") -> (0:w2070:bool)
            n1301 = Select(t="on", s="Trap 2 (ON/OFF)", f="off") -> (s? t:f=w2069:string)
            n1302 = Select(t="on", s="Trap 1 (ON/OFF)", f="off") -> (s? t:f=w2065:string)
            n1303 = Build Array("trap 1 ", w2065) -> (w2064:string[])
            n1304 = Build Array("trap 2 " ("f"), w2069) -> (w2067:string[])
            n1305 = Select(t=w2064, s=w2070, f=w2067) -> (s? t:f=w2063:string[])
            n1306 = property on="Trap 1 ON" class="Bool (strict)"("Val(Sgnl)"="Trap 1 (ON/OFF)") -> ()  [unwired: 2 in, 2 out]
            n1307 = property on="Trap 2 ON" class="Bool (strict)"("Val(Sgnl)"="Trap 2 (ON/OFF)") -> ()  [unwired: 2 in, 2 out]
          }
        }
        n1308 = local read "Saving..."() -> (w2056:bool)
        n1309 = local read "Save Event Log?"() -> (w2055:bool)
        n1310 = And(x=w2056, y=w2055) -> (x .and. y?=w2054:bool)
        n1311 = case shown="True" w2054 {
          tunnel: w2053 -> [_ w2061]
          frame False {
          }
          frame True {
            n1312 = local read "Time (s)"() -> (w2058:dbl)
            n1313 = local read "log file ref"() -> (w2060:refnum<file>)
            n1314 = Concatenate Strings(w2061) -> (w2059:string)
            n1315 = call "write to event log.vi"("log file ref"=w2060, "time"=w2058, "input string"=w2059) -> ()  [unwired: 8 in]
          }
        }
      }
      event "DIO count 1 (ticks)", "DIO count 2 (ticks)", "DIO count 3 (ticks)", "Interlace", "Number Interlace Sets", "Not-Interlacing Set", "BD 1 Delay (ticks)", "BD 2 Delay (Ticks)", "Next trap write delay (ticks)", "Phase offset method", "Phase Increment Trap 1", "Phase Increment Trap 2", "RF phase reset before cycles": Value Change {
        n1316 = event-data() -> ()  [unwired: 7 out]
        n1317 = To Unsigned Byte Integer(number="Not-Interlacing Set") -> (unsigned 8bit integer=w2082:u8)
        n1318 = Add(x=u8 1 ("y"), y=w2082) -> (x+y=w2091:u8)
        n1319 = local read "DIO count 1 (ticks)"() -> (w2098:u16)
        n1320 = local read "DIO count 2 (ticks)"() -> (w2097:u16)
        n1321 = local read "DIO count 3 (ticks)"() -> (w2096:u16)
        n1322 = local read "RF phase reset before cycles"() -> (w2078:bool)
        n1323 = local read "Phase Increment Trap 1"() -> (w2080:fxp<+,14,14>)
        n1324 = local read "Phase offset method"() -> (w2081:u8)
        n1325 = local read "Phase Increment Trap 2"() -> (w2079:fxp<+,14,14>)
        n1326 = xnode "Read/Write Control"("FPGA VI Reference In"=w2084, "DIO count 1 (ticks)"=w2098, "DIO count 2 (ticks)"=w2097, "DIO count 3 (ticks)"=w2096, "Interlace ON/OFF"="Interlace", "Number Interlace Cycles"="Number Interlace Sets", "Interlace Off Parameters"=w2091, "BD 1 Delay (ticks)"="BD 1 Delay (ticks)", "BD 2 Delay (Ticks)"="BD 2 Delay (Ticks)", "Next trap write delay (ticks)"="Next trap write delay (ticks)", "Phase offset method"=w2081, "Phase Trap 1"=w2080, "Phase Trap 2"=w2079, "RF phase reset before cycles"=w2078) -> ("error out"=w2100:errorcluster)  [unwired: 1 in, 1 out]
        n1327 = Build Array(w2098, w2097, w2096) -> (w2090:u16[])
        n1328 = Split 1D Array(array=w2090, index="Number Interlace Sets") -> (first subarray=w2099:u16[])  [unwired: 1 out]
        n1329 = Index Array(array=w2090, index=w2082) -> (element=w2089:u16)
        n1330 = Add Array Elements(numeric array=w2099) -> (sum=w2093:u16)
        n1331 = Select(t=w2093, s="Interlace", f=w2089) -> (s? t:f=→"Total Counts (ticks)":u16)
      }
      event "Reset Feedback": Value Change {
        n1332 = event-data() -> ()  [unwired: 7 out]
        n1333 = Unbundle By Name("Reset Feedback") -> ("Set 1"=w2104:bool, "Set 2"=w2103:bool)
        n1334 = xnode "Read/Write Control"("FPGA VI Reference In"=w2101, "FB Reset Set 1"=w2104, "FB Reset Set 2"=w2103) -> ("error out"=w2102:errorcluster)  [unwired: 1 in, 1 out]
      }
      event "Trap intensity output range", "Trap Intensity PID Gains": Value Change {
        n1335 = event-data() -> ()  [unwired: 7 out]
        n1336 = xnode "Read/Write Control"("FPGA VI Reference In"=w2108, "FB Gains"="Trap Intensity PID Gains", "FB output range"="Trap intensity output range") -> ("error out"=w2109:errorcluster)  [unwired: 1 in, 1 out]
      }
      event "AI2 to Setpoint", "Setpoints (V)": Value Change {
        n1337 = event-data() -> ()  [unwired: 7 out]
        n1338 = xnode "Read/Write Control"("FPGA VI Reference In"=w2110) -> ("FPGA VI Reference Out"=w2113:T41, "error out"=w2112:errorcluster, "AI2 Y Sum Set 1"=w2120:i16, "AI2 Y Sum Set 2"=w2119:i16)  [unwired: 1 in]
        n1339 = Cluster To Array(cluster="AI2 to Setpoint") -> (array=w2123:bool[])
        n1340 = local read "AI2 (V)"() -> (w2121:cluster{"Set 1":dbl, "Set 2":dbl})
        n1341 = Or Array Elements(Boolean array=w2123) -> (logical OR=w2124:bool)
        n1342 = Bundle By Name(cluster=w2121, "Set 1"=w2120, "Set 2"=w2119) -> (w2118:cluster{"Set 1":dbl, "Set 2":dbl})
        n1343 = Divide(x=w2118, y=3276.7) -> (x/y=w2117:cluster{"Set 1":dbl, "Set 2":dbl})
        "AI2 (V)" <- w2117
        n1344 = case shown="True" w2124 {
          tunnel: [w2127 w2144] -> w2116
          tunnel: "AI2 to Setpoint" -> [_ w2140]
          tunnel: "Setpoints (V)" -> [w2128 w2143]
          tunnel: w2117 -> [_ w2137]
          frame False {
            n1345 = Multiply(x=3276.7, y=w2128) -> (x*y=w2129:cluster{"Set 1":dbl, "Set 2":dbl})
            n1346 = To Word Integer(number=w2129) -> (16bit integer=w2127:cluster{"Set 1":i16, "Set 2":i16})
          }
          frame True {
            n1347 = Unbundle By Name(w2137) -> ("Set 1"=w2136:dbl, "Set 2"=w2135:dbl)
            n1348 = Unbundle By Name(w2143) -> ("Set 1"=w2142:dbl, "Set 2"=w2141:dbl)
            n1349 = Unbundle By Name(w2140) -> ("Set 1"=w2139:bool, "Set 2"=w2138:bool)
            n1350 = Select(t=w2136, s=w2139, f=w2142) -> (s? t:f=w2134:dbl)
            n1351 = Select(t=w2135, s=w2138, f=w2141) -> (s? t:f=w2133:dbl)
            n1352 = Bundle By Name(cluster=w2143, "Set 1"=w2134, "Set 2"=w2133) -> (w2131:cluster{"Set 1":dbl, "Set 2":dbl})
            n1353 = local write "Setpoints (V)"(w2131) -> ()
            n1354 = Multiply(x=3276.7, y=w2131) -> (x*y=w2132:cluster{"Set 1":dbl, "Set 2":dbl})
            n1355 = To Word Integer(number=w2132) -> (16bit integer=w2144:cluster{"Set 1":i16, "Set 2":i16})
          }
        }
        n1356 = Unbundle By Name(w2116) -> ("Set 1"=w2115:i16, "Set 2"=w2114:i16)
        n1357 = xnode "Read/Write Control"("FPGA VI Reference In"=w2113, "error in"=w2112, "FB Setpoint Set 1"=w2115, "FB Setpoint Set 2"=w2114) -> ("error out"=w2111:errorcluster)  [unwired: 1 out]
      }
      event "+ phase (Vortran)", "- phase (Vortran)", "+ phase (GI) 2", "- phase (GI) 2", "+ phase (RI)", "- phase (RI)", "+ phase (Green FB)", "- phase (Green FB)", "- phase (BI AO)", "+ phase (BI AO)", "- phase (BI DO)", "+ phase (BI DO)": Value Change {
        n1358 = event-data() -> ()  [unwired: 7 out]
        n1359 = Or(x="+ phase (Vortran)", y="- phase (Vortran)") -> (x .or. y?=w2180:bool)
        n1360 = Negate(x="Phase adj. (Vortran)") -> (-x=w2185:i16)
        n1361 = Select(t=w2185, s="+ phase (Vortran)", f="Phase adj. (Vortran)") -> (s? t:f=w2184:i16)
        n1362 = Or(x="+ phase (GI) 2", y="- phase (GI) 2") -> (x .or. y?=w2171:bool)
        n1363 = Negate(x="Phase adj. (GI) 2") -> (-x=w2176:i16)
        n1364 = Select(t=w2176, s="+ phase (GI) 2", f="Phase adj. (GI) 2") -> (s? t:f=w2172:i16)
        n1365 = Negate(x="Phase adj. (RI)") -> (-x=w2170:i16)
        n1366 = Or(x="+ phase (RI)", y="- phase (RI)") -> (x .or. y?=w2166:bool)
        n1367 = Select(t=w2170, s="+ phase (RI)", f="Phase adj. (RI)") -> (s? t:f=w2165:i16)
        n1368 = Or(x="+ phase (Green FB)", y="- phase (Green FB)") -> (x .or. y?=w2159:bool)
        n1369 = Negate(x="Phase adj. (Green FB)") -> (-x=w2164:i16)
        n1370 = Select(t=w2164, s="+ phase (Green FB)", f="Phase adj. (Green FB)") -> (s? t:f=w2160:i16)
        n1371 = Negate(x="Phase adj. (BI AO)") -> (-x=w2158:i16)
        n1372 = Or(x="+ phase (BI AO)", y="- phase (BI AO)") -> (x .or. y?=w2148:bool)
        n1373 = Select(t=w2158, s="+ phase (BI AO)", f="Phase adj. (BI AO)") -> (s? t:f=w2150:i16)
        n1374 = Negate(x="Phase adj. (BI DO)") -> (-x=w2154:i16)
        n1375 = Or(x="+ phase (BI DO)", y="- phase (BI DO)") -> (x .or. y?=w2147:bool)
        n1376 = Select(t=w2154, s="+ phase (BI DO)", f="Phase adj. (BI DO)") -> (s? t:f=w2149:i16)
        n1377 = xnode "Read/Write Control"("FPGA VI Reference In"=w2146, "Phase count adjustment (GI)"=w2184, "Phase count adjustment (GI) 2"=w2172, "Phase count adjustment (RI)"=w2165, "Phase count adjustment (Green FB)"=w2160, "Phase count adjustment (BI AO)"=w2150, "Phase count adjustment (BI D)"=w2149) -> ("FPGA VI Reference Out"=w2182:T41, "error out"=w2183:errorcluster)  [unwired: 1 in]
        n1378 = xnode "Read/Write Control"("FPGA VI Reference In"=w2182, "error in"=w2183, "+ phase (GI)"=w2180, "+ phase (GI) 2"=w2171, "+ phase (RI)"=w2166, "+ phase (Green FB)"=w2159, "+ phase (BI AO)"=w2148, "+ phase (BI D)"=w2147) -> ("error out"=w2181:errorcluster)  [unwired: 1 out]
      }
      event "Green Laser ON/OFF", "Red Laser ON/OFF", "Blue Laser ON/OFF": Value Change {
        # "This loop shouldn't be initialized.  The main 'laser ON' settings should dominate and set the others."
        n1379 = event-data() -> ()  [unwired: 7 out]
        n1380 = property on="Red Laser ON" class="Bool (strict)"("Val(Sgnl)"="Red Laser ON/OFF") -> ()  [unwired: 2 in, 2 out]
        n1381 = property on="Blue Laser ON" class="Bool (strict)"("Val(Sgnl)"="Blue Laser ON/OFF") -> ()  [unwired: 2 in, 2 out]
        n1382 = property on="Vortran Laser ON" class="Bool (strict)"("Val(Sgnl)"="Green Laser ON/OFF") -> ()  [unwired: 2 in, 2 out]
      }
      event "Laser interlacing mode", "Vortran Laser ON", "Red Laser ON", "Blue Laser ON": Value Change {
        n1383 = event-data() -> ()  [unwired: 7 out]
        n1384 = local write "Green Laser ON/OFF"("Vortran Laser ON") -> ()
        n1385 = local write "Blue Laser ON/OFF"("Blue Laser ON") -> ()
        n1386 = local write "Red Laser ON/OFF"("Red Laser ON") -> ()